vi "SO2 ZeroAir Gas Preparation.vi"() -> ()   [LabVIEW 2014]
panel:
  out "CO preflight Des 1":string="SO2 Ground ZeroAir Gas Preflight Checks - DO NOT GET DISTRACTED!\n\n1. Check quick connect male body is connected to 'chem 2' gas line.\n\n2. Back out (V2) delivery control valve (anticlockwise).\n\n3. Open cylinder valve V1.\n\n4. Set regulator (V2) to deliver at 3 bar (clockwise).\n\n5. Note cylinder content pressure in chemistry e-Log.\n"
  in  "Exit":bool
  # "V2"
  # "V1"
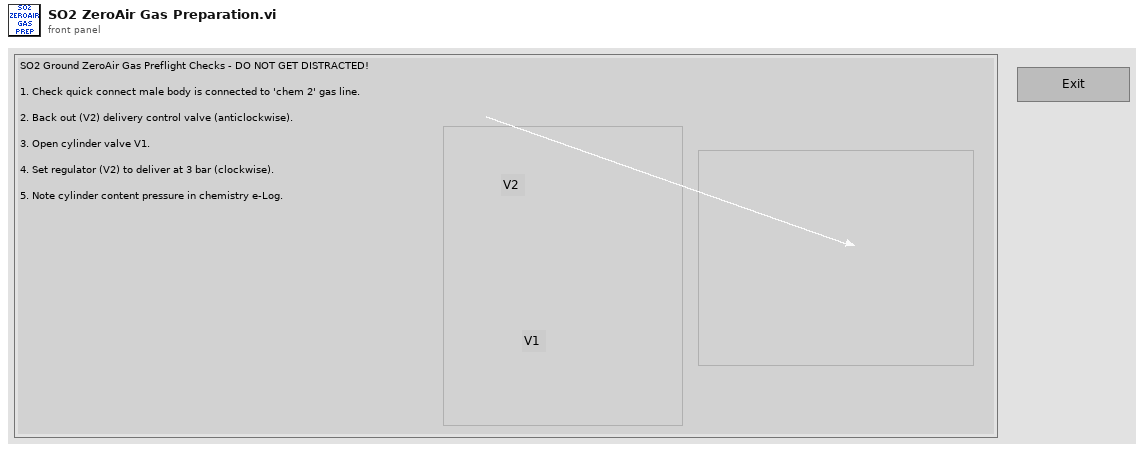
[diagram p1: front panel]
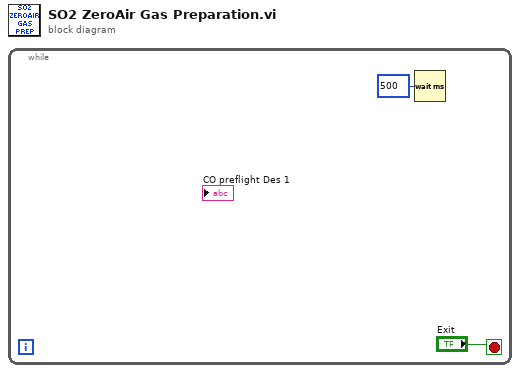
[diagram p0: block diagram]
diagram:
  n1 = while {
    stop <- "Exit" stop-if-true
    n2 = Wait (ms)(milliseconds to wait=u32 500) -> ()  [unwired: 1 out]
  }
